vi "TLB Native Dynamic Events ver 0.25.vi"() -> ()   [LabVIEW 2018] (continued)
            n517 = Less?(x=w1477, y=w1481) -> (x < y?=w1480:bool)
            n518 = And(x=w1480, y=w1479) -> (x .and. y?=w1476:bool)
            n519 = case shown="\"Start Task 1\", Default" w1483 {
              tunnel: [w1498 State_Type_Definitions."True Stop" ("Enum")] -> w1488
              tunnel: [w1501 w1518] -> w1487
              tunnel: [State_Type_Definitions."Idle" ("Enum") State_Type_Definitions."Shutdown" ("Enum")] -> w1489
              tunnel: w1491 -> [w1497 _]
              tunnel: w1490 -> [w1493 w1515]
              tunnel: w1476 -> [w1492 _]
              frame "Start Task 1", Default {
                # "Stays in Task 5_B to capture image over 5 seconds"
                # "T: Go back to idle, F: Continue with task\""
                # ">> Manual override >>"
                n520 = case shown="True" w1492 {
                  tunnel: [w1505 w1511] -> w1501
                  tunnel: w1493 -> [w1503 w1509]
                  frame False {
                    n521 = for {
                      tunnel: string[] ["FORWARD", "READ ULTRASONIC", "READ NAVX"] ("element") -> [w1506] mode=indexing
                      shift-right: [w1508] -> w1505
                      shift-left: w1503 -> [w1507]
                      n522 = Enqueue Element(queue=w1507, element=w1506) -> (queue out=w1508:refnum<queue>)  [unwired: 2 in, 2 out]
                    }
                  }
                  frame True {
                    n523 = for {
                      shift-right: [w1513] -> w1511
                      shift-left: w1509 -> [w1514]
                      tunnel: string[] ["STOP", "RESET ENCODERS", "OPEN LOG CAM", "SET TIMER 2", "OPEN IMAQ REF"] -> [w1512] mode=indexing
                      n524 = Enqueue Element(queue=w1514, element=w1512) -> (queue out=w1513:refnum<queue>)  [unwired: 2 in, 2 out]
                    }
                  }
                }
                n525 = Or(x=w1492, y=w1497) -> (x .or. y?=w1499:bool)
                n526 = Select(t=State_Type_Definitions."True Stop" ("Enum"), s=w1497, f=State_Type_Definitions."Task 8C: CAM BURST" ("Enum")) -> (s? t:f=w1494:T16)
                n527 = Select(t=w1494, s=w1499, f=State_Type_Definitions."Task 8B: MOVE TO BOX" ("Enum")) -> (s? t:f=w1498:T16)
              }
              frame "Exit" {
                n528 = for {
                  shift-right: [w1521] -> w1518
                  shift-left: w1515 -> [w1522]
                  tunnel: string[] ["STOP", "RESET ENCODERS", "RESET YAW", "ARDUINO MODE 0"] -> [w1520] mode=indexing
                  n529 = Enqueue Element(queue=w1522, element=w1520) -> (queue out=w1521:refnum<queue>)  [unwired: 2 in, 2 out]
                }
              }
            }
          }
          frame "Task 8C: CAM BURST" {
            # ">>> Motor control cluster >>>"
            # ">>> yStepper command>>>"
            # ">> Manual override >>"
            n530 = Dequeue Element(queue=w1533, timeout in ms (-1)=w1532, error in (no error)=w1531) -> (element=w1530:T8)  [unwired: 3 out]
            n531 = case shown="\"Start Task 1\", Default" w1530 {
              tunnel: [w1542 State_Type_Definitions."True Stop" ("Enum")] -> w1535
              tunnel: [w1545 w1562] -> w1528
              tunnel: [State_Type_Definitions."Idle" ("Enum") State_Type_Definitions."Shutdown" ("Enum")] -> w1527
              tunnel: w1529 -> [w1536 _]
              tunnel: w1534 -> [w1541 w1559]
              tunnel: w1525 -> [w1540 _]
              frame "Start Task 1", Default {
                # ">> Is time up? >>"
                # "Determines if object is in range to pick up"
                # ">> Manual override >>"
                n532 = case shown="True" w1540 {
                  tunnel: [w1549 w1555] -> w1545
                  tunnel: w1541 -> [w1547 w1553]
                  frame False {
                    n533 = for {
                      tunnel: string[] ["CAM ACQ", "START TIMER"] ("element") -> [w1550] mode=indexing
                      shift-right: [w1552] -> w1549
                      shift-left: w1547 -> [w1551]
                      n534 = Enqueue Element(queue=w1551, element=w1550) -> (queue out=w1552:refnum<queue>)  [unwired: 2 in, 2 out]
                    }
                  }
                  frame True {
                    n535 = for {
                      shift-right: [w1557] -> w1555
                      shift-left: w1553 -> [w1558]
                      tunnel: string[] ["CAM CLOSE", "PROCESS IMAGE", "SET TIMER 5"] -> [w1556] mode=indexing
                      n536 = Enqueue Element(queue=w1558, element=w1556) -> (queue out=w1557:refnum<queue>)  [unwired: 2 in, 2 out]
                    }
                  }
                }
                n537 = Or(x=w1540, y=w1536) -> (x .or. y?=w1543:bool)
                n538 = Select(t=State_Type_Definitions."True Stop" ("Enum"), s=w1536, f=State_Type_Definitions."Task 8D: PROCESS IMAGE" ("Enum")) -> (s? t:f=w1538:T16)
                n539 = Select(t=w1538, s=w1543, f=State_Type_Definitions."Task 8C: CAM BURST" ("Enum")) -> (s? t:f=w1542:T16)
              }
              frame "Exit" {
                n540 = for {
                  shift-right: [w1565] -> w1562
                  shift-left: w1559 -> [w1566]
                  tunnel: string[] ["STOP", "RESET ENCODERS", "RESET YAW", "ARDUINO MODE 0"] -> [w1564] mode=indexing
                  n541 = Enqueue Element(queue=w1566, element=w1564) -> (queue out=w1565:refnum<queue>)  [unwired: 2 in, 2 out]
                }
              }
            }
          }
          frame "Task 8D: PROCESS IMAGE" {
            # ">>> yStepper command>>>"
            n542 = Dequeue Element(queue=w1574, timeout in ms (-1)=w1573, error in (no error)=w1572) -> (element=w1571:T8)  [unwired: 3 out]
            n543 = case shown="\"Start Task 1\", Default" w1571 {
              tunnel: [w1586 State_Type_Definitions."True Stop" ("Enum")] -> w1578
              tunnel: [w1589 w1606] -> w1577
              tunnel: [State_Type_Definitions."Idle" ("Enum") State_Type_Definitions."Shutdown" ("Enum")] -> w1579
              tunnel: w1575 -> [w1585 _]
              tunnel: w1576 -> [w1581 w1603]
              tunnel: w1569 -> [w1580 _]
              frame "Start Task 1", Default {
                # ">> T: Breaks out of state loop; F: Stays in loop>>"
                # ">> Manual override >>"
                # ">> Checks if time is up>>"
                # "Stays in Task 5D until the object is detected"
                # "T: Go back to idle, F: Continue with task\""
                # ">> Manual override >>"
                n544 = case shown="True" w1580 {
                  tunnel: [w1593 w1599] -> w1589
                  tunnel: w1581 -> [w1591 w1597]
                  frame False {
                    n545 = for {
                      tunnel: string[] ["START TIMER", "PROCESS IMAGE", ""] ("element") -> [w1594] mode=indexing
                      shift-right: [w1596] -> w1593
                      shift-left: w1591 -> [w1595]
                      n546 = Enqueue Element(queue=w1595, element=w1594) -> (queue out=w1596:refnum<queue>)  [unwired: 2 in, 2 out]
                    }
                  }
                  frame True {
                    n547 = for {
                      shift-right: [w1601] -> w1599
                      shift-left: w1597 -> [w1602]
                      tunnel: string[] ["RESET ENCODERS", "", ""] -> [w1600] mode=indexing
                      n548 = Enqueue Element(queue=w1602, element=w1600) -> (queue out=w1601:refnum<queue>)  [unwired: 2 in, 2 out]
                    }
                  }
                }
                n549 = Or(x=w1580, y=w1585) -> (x .or. y?=w1587:bool)
                n550 = Select(t=State_Type_Definitions."True Stop" ("Enum"), s=w1585, f=State_Type_Definitions."Task 8E: ROBOT ADJUST" ("Enum")) -> (s? t:f=w1582:T16)
                n551 = Select(t=w1582, s=w1587, f=State_Type_Definitions."Task 8D: PROCESS IMAGE" ("Enum")) -> (s? t:f=w1586:T16)
              }
              frame "Exit" {
                n552 = for {
                  shift-right: [w1609] -> w1606
                  shift-left: w1603 -> [w1610]
                  tunnel: string[] ["STOP", "RESET ENCODERS", "RESET YAW", "ARDUINO MODE 0"] -> [w1608] mode=indexing
                  n553 = Enqueue Element(queue=w1610, element=w1608) -> (queue out=w1609:refnum<queue>)  [unwired: 2 in, 2 out]
                }
              }
            }
          }
          frame "Task 8E: ROBOT ADJUST" {
            # ">>> Motor control cluster >>>"
            # ">>> yStepper command>>>"
            n554 = Dequeue Element(queue=w1627, timeout in ms (-1)=w1626, error in (no error)=w1625) -> (element=w1624:T8)  [unwired: 3 out]
            n555 = Subtract(x=w1622, y=300.0) -> (x-y=w1620:dbl)
            n556 = formula code="if (error <= -61&&error > -300){\ndistance = -15;\nxSpeed = -30;\n}\n\nelse if (error <= -51 && error >= -60){\ndistance = -10;\nxSpeed = -30;\n}\n\nelse if (error >= -50 && error <= 50){\ndistance = 0;\nxSpeed = 0;\n}\n\nelse if (error >= 51 && error <= 80){\ndistance = 10;\nxSpeed = 30;\n}\n\nelse if (error >= 81 && error <= 100){\ndistance = 15;\nxSpeed = 30;\n}\n\nelse if (error >= 101 && error <= 120){\ndistance = 20;\nxSpeed = 30;\n}\n\nelse if (error >= 121 && error < 300){\ndistance = 25;\nxSpeed = 30;\n}\n\nelse{\ndistance = 0;\nxSpeed = 0;\n}"("error"=w1620) -> ("distance"=w1615:dbl, "xSpeed"=w1617:dbl)
            n557 = formula code="if (target > 0){\nif (current  >= target)\noutput = 1;\n\nelse if (current != target)\noutput = 0;\n}\n\nelse if (target == 0){\nif (current == target)\noutput = 1;\n\nelse if (current != target)\noutput = 0;\n}\n\nelse if (target < 0){\nif (current <= target)\noutput = 1;\n\nelse if (current != target)\noutput = 0;\n}\n\nelse if (current != target)\noutput = 0;"("target"=w1615, "current"=w1616) -> ("output"=w1614:dbl)
            n558 = Bundle By Name(cluster=w1619, "xSpeed"=w1617) -> (w1618:T17)
            n559 = Equal?(x=w1614, y=1.0) -> (x = y?=w1612:bool)
            n560 = case shown="\"Start Task 1\", Default" w1624 {
              tunnel: [w1639 State_Type_Definitions."True Stop" ("Enum")] -> w1631
              tunnel: [w1642 w1659] -> w1630
              tunnel: [State_Type_Definitions."Idle" ("Enum") State_Type_Definitions."Shutdown" ("Enum")] -> w1632
              tunnel: w1628 -> [w1638 _]
              tunnel: w1629 -> [w1634 w1656]
              tunnel: w1612 -> [w1633 _]
              frame "Start Task 1", Default {
                # ">> T: Breaks out of state loop; F: Stays in loop>>"
                # ">> Manual override >>"
                # ">> Checks if time is up>>"
                # "Stays in Task 5D until the object is detected"
                # "T: Go back to idle, F: Continue with task\""
                # ">> Manual override >>"
                n561 = case shown="True" w1633 {
                  tunnel: [w1646 w1652] -> w1642
                  tunnel: w1634 -> [w1644 w1650]
                  frame False {
                    n562 = for {
                      tunnel: string[] ["X AXIS - SLOW", "READ ENCODERS", "READ NAVX"] ("element") -> [w1647] mode=indexing
                      shift-right: [w1649] -> w1646
                      shift-left: w1644 -> [w1648]
                      n563 = Enqueue Element(queue=w1648, element=w1647) -> (queue out=w1649:refnum<queue>)  [unwired: 2 in, 2 out]
                    }
                  }
                  frame True {
                    n564 = for {
                      shift-right: [w1654] -> w1652
                      shift-left: w1650 -> [w1655]
                      tunnel: string[] ["SET TIMER 2", "STOP", "READ STEPPER VALUES", ""] -> [w1653] mode=indexing
                      n565 = Enqueue Element(queue=w1655, element=w1653) -> (queue out=w1654:refnum<queue>)  [unwired: 2 in, 2 out]
                    }
                  }
                }
                n566 = Or(x=w1633, y=w1638) -> (x .or. y?=w1640:bool)
                n567 = Select(t=State_Type_Definitions."True Stop" ("Enum"), s=w1638, f=State_Type_Definitions."Task 8H: ARM ADJUST" ("Enum")) -> (s? t:f=w1635:T16)
                n568 = Select(t=w1635, s=w1640, f=State_Type_Definitions."Task 8E: ROBOT ADJUST" ("Enum")) -> (s? t:f=w1639:T16)
              }
              frame "Exit" {
                n569 = for {
                  shift-right: [w1662] -> w1659
                  shift-left: w1656 -> [w1663]
                  tunnel: string[] ["STOP", "RESET ENCODERS", "RESET YAW", "ARDUINO MODE 0"] -> [w1661] mode=indexing
                  n570 = Enqueue Element(queue=w1663, element=w1661) -> (queue out=w1662:refnum<queue>)  [unwired: 2 in, 2 out]
                }
              }
            }
          }
          frame "Task 8F: CAM BURST 2" {
            # ">>> Motor control cluster >>>"
            # ">>> yStepper command>>>"
            # ">> Manual override >>"
            n571 = Dequeue Element(queue=w1674, timeout in ms (-1)=w1673, error in (no error)=w1672) -> (element=w1671:T8)  [unwired: 3 out]
            n572 = case shown="\"Start Task 1\", Default" w1671 {
              tunnel: [w1683 State_Type_Definitions."True Stop" ("Enum")] -> w1676
              tunnel: [w1686 w1703] -> w1669
              tunnel: [State_Type_Definitions."Idle" ("Enum") State_Type_Definitions."Shutdown" ("Enum")] -> w1668
              tunnel: w1670 -> [w1677 _]
              tunnel: w1675 -> [w1682 w1700]
              tunnel: w1666 -> [w1681 _]
              frame "Start Task 1", Default {
                # ">> Is time up? >>"
                # "Determines if object is in range to pick up"
                # ">> Manual override >>"
                n573 = case shown="False" w1681 {
                  tunnel: [w1690 w1696] -> w1686
                  tunnel: w1682 -> [w1688 w1694]
                  frame False {
                    n574 = for {
                      tunnel: string[] ["CAM ACQ", "START TIMER"] ("element") -> [w1691] mode=indexing
                      shift-right: [w1693] -> w1690
                      shift-left: w1688 -> [w1692]
                      n575 = Enqueue Element(queue=w1692, element=w1691) -> (queue out=w1693:refnum<queue>)  [unwired: 2 in, 2 out]
                    }
                  }
                  frame True {
                    n576 = for {
                      shift-right: [w1698] -> w1696
                      shift-left: w1694 -> [w1699]
                      tunnel: string[] ["CAM CLOSE", "PROCESS IMAGE", "SET TIMER 3"] -> [w1697] mode=indexing
                      n577 = Enqueue Element(queue=w1699, element=w1697) -> (queue out=w1698:refnum<queue>)  [unwired: 2 in, 2 out]
                    }
                  }
                }
                n578 = Or(x=w1681, y=w1677) -> (x .or. y?=w1684:bool)
                n579 = Select(t=State_Type_Definitions."True Stop" ("Enum"), s=w1677, f=State_Type_Definitions."Task 8G: PROCESS IMAGE 2" ("Enum")) -> (s? t:f=w1679:T16)
                n580 = Select(t=w1679, s=w1684, f=State_Type_Definitions."Task 8F: CAM BURST 2" ("Enum")) -> (s? t:f=w1683:T16)
              }
              frame "Exit" {
                n581 = for {
                  shift-right: [w1706] -> w1703
                  shift-left: w1700 -> [w1707]
                  tunnel: string[] ["STOP", "RESET ENCODERS", "RESET YAW", "ARDUINO MODE 0"] -> [w1705] mode=indexing
                  n582 = Enqueue Element(queue=w1707, element=w1705) -> (queue out=w1706:refnum<queue>)  [unwired: 2 in, 2 out]
                }
              }
            }
          }
          frame "Task 8G: PROCESS IMAGE 2" {
            # ">>> yStepper command>>>"
            n583 = Dequeue Element(queue=w1715, timeout in ms (-1)=w1714, error in (no error)=w1713) -> (element=w1712:T8)  [unwired: 3 out]
            n584 = case shown="\"Start Task 1\", Default" w1712 {
              tunnel: [w1727 State_Type_Definitions."True Stop" ("Enum")] -> w1719
              tunnel: [w1730 w1747] -> w1718
              tunnel: [State_Type_Definitions."Idle" ("Enum") State_Type_Definitions."Shutdown" ("Enum")] -> w1720
              tunnel: w1716 -> [w1726 _]
              tunnel: w1717 -> [w1722 w1744]
              tunnel: w1710 -> [w1721 _]
              frame "Start Task 1", Default {
                # ">> T: Breaks out of state loop; F: Stays in loop>>"
                # ">> Manual override >>"
                # ">> Checks if time is up>>"
                # "Stays in Task 5D until the object is detected"
                # "T: Go back to idle, F: Continue with task\""
                # ">> Manual override >>"
                n585 = case shown="False" w1721 {
                  tunnel: [w1734 w1740] -> w1730
                  tunnel: w1722 -> [w1732 w1738]
                  frame False {
                    n586 = for {
                      tunnel: string[] ["START TIMER", "PROCESS IMAGE", ""] ("element") -> [w1735] mode=indexing
                      shift-right: [w1737] -> w1734
                      shift-left: w1732 -> [w1736]
                      n587 = Enqueue Element(queue=w1736, element=w1735) -> (queue out=w1737:refnum<queue>)  [unwired: 2 in, 2 out]
                    }
                  }
                  frame True {
                    n588 = for {
                      shift-right: [w1742] -> w1740
                      shift-left: w1738 -> [w1743]
                      tunnel: string[] ["READ STEPPER VALUES", "Y STEPPER CONTROL", ""] -> [w1741] mode=indexing
                      n589 = Enqueue Element(queue=w1743, element=w1741) -> (queue out=w1742:refnum<queue>)  [unwired: 2 in, 2 out]
                    }
                  }
                }
                n590 = Or(x=w1721, y=w1726) -> (x .or. y?=w1728:bool)
                n591 = Select(t=State_Type_Definitions."True Stop" ("Enum"), s=w1726, f=State_Type_Definitions."Task 8H: ARM ADJUST" ("Enum")) -> (s? t:f=w1723:T16)
                n592 = Select(t=w1723, s=w1728, f=State_Type_Definitions."Task 8G: PROCESS IMAGE 2" ("Enum")) -> (s? t:f=w1727:T16)
              }
              frame "Exit" {
                n593 = for {
                  shift-right: [w1750] -> w1747
                  shift-left: w1744 -> [w1751]
                  tunnel: string[] ["STOP", "RESET ENCODERS", "RESET YAW", "ARDUINO MODE 0"] -> [w1749] mode=indexing
                  n594 = Enqueue Element(queue=w1751, element=w1749) -> (queue out=w1750:refnum<queue>)  [unwired: 2 in, 2 out]
                }
              }
            }
          }
          frame "Task 8H: ARM ADJUST" {
            # ">>> yStepper command>>>"
            n595 = Dequeue Element(queue=w1765, timeout in ms (-1)=w1766, error in (no error)=w1767) -> (element=w1769:T8)  [unwired: 3 out]
            n596 = formula code="if (pos < 70)\ny = 43;\n\nelse if (pos >= 71 &&pos <= 80)\ny = 40;\n\nelse if (pos >= 81 && pos <= 90)\ny = 38;\n\nelse if (pos >= 91 &&pos <= 120)\ny = 35;\n\nelse if (pos >= 121 && pos <= 140)\ny = 30;\n\nelse if (pos >= 141 && pos <= 170)\ny = 26;\n\nelse if (pos >= 171 &&pos <= 220) \ny = 20;\n\nelse if (pos >= 221&& pos <= 240)\ny = 15;\n\nelse if (pos >= 241 && pos <= 250)\ny = 10;\n\nelse if (pos >= 251)\ny = 0;"("pos"=w1757) -> ("y"=w1760:dbl)
            n597 = To Unsigned Byte Integer(number=w1760) -> (unsigned 8bit integer=w1755:u8)
            n598 = Equal?(x=w1756, y=w1755) -> (x = y?=w1754:bool)
            n599 = case shown="\"Start Task 1\", Default" w1769 {
              tunnel: [w1776 State_Type_Definitions."True Stop" ("Enum")] -> w1763
              tunnel: [w1779 w1796] -> w1761
              tunnel: [State_Type_Definitions."Idle" ("Enum") State_Type_Definitions."Shutdown" ("Enum")] -> w1762
              tunnel: w1768 -> [w1775 _]
              tunnel: w1764 -> [w1771 w1793]
              tunnel: w1754 -> [w1770 _]
              frame "Start Task 1", Default {
                # ">> T: Breaks out of state loop; F: Stays in loop>>"
                # ">> Manual override >>"
                # ">> Checks if time is up>>"
                # "Stays in Task 5D until the object is detected"
                # "T: Go back to idle, F: Continue with task\""
                # ">> Manual override >>"
                n600 = case shown="False" w1770 {
                  tunnel: [w1783 w1789] -> w1779
                  tunnel: w1771 -> [w1781 w1787]
                  frame False {
                    n601 = for {
                      tunnel: string[] ["READ STEPPER VALUES", "Y STEPPER CONTROL", ""] ("element") -> [w1784] mode=indexing
                      shift-right: [w1786] -> w1783
                      shift-left: w1781 -> [w1785]
                      n602 = Enqueue Element(queue=w1785, element=w1784) -> (queue out=w1786:refnum<queue>)  [unwired: 2 in, 2 out]
                    }
                  }
                  frame True {
                    n603 = for {
                      shift-right: [w1791] -> w1789
                      shift-left: w1787 -> [w1792]
                      tunnel: string[] ["DISPOSE BUFFERS", "READ STEPPER VALUES", ""] -> [w1790] mode=indexing
                      n604 = Enqueue Element(queue=w1792, element=w1790) -> (queue out=w1791:refnum<queue>)  [unwired: 2 in, 2 out]
                    }
                  }
                }
                n605 = Or(x=w1770, y=w1775) -> (x .or. y?=w1777:bool)
                n606 = Select(t=State_Type_Definitions."True Stop" ("Enum"), s=w1775, f=State_Type_Definitions."Task 8I: ARM GRAB HEIGHT" ("Enum")) -> (s? t:f=w1772:T16)
                n607 = Select(t=w1772, s=w1777, f=State_Type_Definitions."Task 8H: ARM ADJUST" ("Enum")) -> (s? t:f=w1776:T16)
              }
              frame "Exit" {
                n608 = for {
                  shift-right: [w1799] -> w1796
                  shift-left: w1793 -> [w1800]
                  tunnel: string[] ["STOP", "RESET ENCODERS", "RESET YAW", "ARDUINO MODE 0"] -> [w1798] mode=indexing
                  n609 = Enqueue Element(queue=w1800, element=w1798) -> (queue out=w1799:refnum<queue>)  [unwired: 2 in, 2 out]
                }
              }
            }
            n610 = Bundle By Name(cluster=w1759, "yStepper desired"=w1755) -> (w1758:T18)
          }
          frame "Task 8I: ARM GRAB HEIGHT" {
            # ">>> Motor control cluster >>>"
            # ">>> yStepper command>>>"
            # ">> Manual override >>"
            n611 = Dequeue Element(queue=w1811, timeout in ms (-1)=w1810, error in (no error)=w1812) -> (element=w1809:T8)  [unwired: 3 out]
            n612 = Equal?(x=w1808, y=u8 1) -> (x = y?=w1806:bool)
            n613 = case shown="\"Start Task 1\", Default" w1809 {
              tunnel: [w1822 State_Type_Definitions."True Stop" ("Enum")] -> w1813
              tunnel: [w1825 w1842] -> w1814
              tunnel: [State_Type_Definitions."Idle" ("Enum") State_Type_Definitions."Shutdown" ("Enum")] -> w1815
              tunnel: w1806 -> [w1821 _]
              tunnel: w1805 -> [w1820 _]
              tunnel: w1804 -> [w1816 w1839]
              frame "Start Task 1", Default {
                # "Stays in Task 5F until stepper reaches desired \nheight"
                # "T: Go back to idle, F: Continue with task\""
                # ">> Manual override >>"
                n614 = case shown="True" w1821 {
                  tunnel: [w1829 w1835] -> w1825
                  tunnel: w1816 -> [w1827 w1833]
                  frame False {
                    n615 = for {
                      tunnel: string[] ["Z STEPPER GRAB HEIGHT", "READ STEPPER VALUES"] ("element") -> [w1830] mode=indexing
                      shift-right: [w1832] -> w1829
                      shift-left: w1827 -> [w1831]
                      n616 = Enqueue Element(queue=w1831, element=w1830) -> (queue out=w1832:refnum<queue>)  [unwired: 2 in, 2 out]
                    }
                  }
                  frame True {
                    n617 = for {
                      shift-right: [w1837] -> w1835
                      shift-left: w1833 -> [w1838]
                      tunnel: string[] ["SET TIMER 2", "CLOSE CLAW", ""] -> [w1836] mode=indexing
                      n618 = Enqueue Element(queue=w1838, element=w1836) -> (queue out=w1837:refnum<queue>)  [unwired: 2 in, 2 out]
                    }
                  }
                }
                n619 = Or(x=w1821, y=w1820) -> (x .or. y?=w1823:bool)
                n620 = Select(t=State_Type_Definitions."True Stop" ("Enum"), s=w1820, f=State_Type_Definitions."Task 8J: CLOSE CLAW" ("Enum")) -> (s? t:f=w1817:T16)
                n621 = Select(t=w1817, s=w1823, f=State_Type_Definitions."Task 8I: ARM GRAB HEIGHT" ("Enum")) -> (s? t:f=w1822:T16)
              }
              frame "Exit" {
                n622 = for {
                  shift-right: [w1845] -> w1842
                  shift-left: w1839 -> [w1846]
                  tunnel: string[] ["STOP", "RESET ENCODERS", "RESET YAW", "ARDUINO MODE 0"] -> [w1844] mode=indexing
                  n623 = Enqueue Element(queue=w1846, element=w1844) -> (queue out=w1845:refnum<queue>)  [unwired: 2 in, 2 out]
                }
              }
            }
          }
          frame "Task 8J: CLOSE CLAW" {
            # ">>> yStepper command>>>"
            # ">> Manual override >>"
            n624 = Dequeue Element(queue=w1857, timeout in ms (-1)=w1856, error in (no error)=w1855) -> (element=w1854:T8)  [unwired: 3 out]
            n625 = case shown="\"Start Task 1\", Default" w1854 {
              tunnel: [w1866 State_Type_Definitions."True Stop" ("Enum")] -> w1859
              tunnel: [w1869 w1886] -> w1852
              tunnel: [State_Type_Definitions."Idle" ("Enum") State_Type_Definitions."Shutdown" ("Enum")] -> w1851
              tunnel: w1853 -> [w1860 _]
              tunnel: w1858 -> [w1865 w1883]
              tunnel: w1849 -> [w1864 _]
              frame "Start Task 1", Default {
                # ">> Is time up? >>"
                # "Determines if object is in range to pick up"
                # ">> Manual override >>"
                n626 = case shown="True" w1864 {
                  tunnel: [w1873 w1879] -> w1869
                  tunnel: w1865 -> [w1871 w1877]
                  frame False {
                    n627 = for {
                      tunnel: string[] ["CLOSE CLAW", "START TIMER"] ("element") -> [w1874] mode=indexing
                      shift-right: [w1876] -> w1873
                      shift-left: w1871 -> [w1875]
                      n628 = Enqueue Element(queue=w1875, element=w1874) -> (queue out=w1876:refnum<queue>)  [unwired: 2 in, 2 out]
                    }
                  }
                  frame True {
                    n629 = for {
                      shift-right: [w1881] -> w1879
                      shift-left: w1877 -> [w1882]
                      tunnel: string[] ["READ STEPPER VALUES", "", ""] -> [w1880] mode=indexing
                      n630 = Enqueue Element(queue=w1882, element=w1880) -> (queue out=w1881:refnum<queue>)  [unwired: 2 in, 2 out]
                    }
                  }
                }
                n631 = Or(x=w1864, y=w1860) -> (x .or. y?=w1867:bool)
                n632 = Select(t=State_Type_Definitions."True Stop" ("Enum"), s=w1860, f=State_Type_Definitions."Task 8K: RAISE MY SWORD" ("Enum")) -> (s? t:f=w1862:T16)
                n633 = Select(t=w1862, s=w1867, f=State_Type_Definitions."Task 8J: CLOSE CLAW" ("Enum")) -> (s? t:f=w1866:T16)
              }
              frame "Exit" {
                n634 = for {
                  shift-right: [w1889] -> w1886
                  shift-left: w1883 -> [w1890]
                  tunnel: string[] ["STOP", "RESET ENCODERS", "RESET YAW", "ARDUINO MODE 0"] -> [w1888] mode=indexing
                  n635 = Enqueue Element(queue=w1890, element=w1888) -> (queue out=w1889:refnum<queue>)  [unwired: 2 in, 2 out]
                }
              }
            }
          }
          frame "Task 8K: RAISE MY SWORD" {
            # ">>> yStepper command>>>"
            # ">> Manual override >>"
            n636 = Dequeue Element(queue=w1901, timeout in ms (-1)=w1900, error in (no error)=w1902) -> (element=w1899:T8)  [unwired: 3 out]
            n637 = Equal?(x=w1898, y=u8 60) -> (x = y?=w1896:bool)
            n638 = case shown="\"Start Task 1\", Default" w1899 {
              tunnel: [w1912 State_Type_Definitions."True Stop" ("Enum")] -> w1903
              tunnel: [w1915 w1932] -> w1904
              tunnel: [State_Type_Definitions."Idle" ("Enum") State_Type_Definitions."Shutdown" ("Enum")] -> w1905
              tunnel: w1896 -> [w1911 _]
              tunnel: w1895 -> [w1910 _]
              tunnel: w1894 -> [w1906 w1929]
              frame "Start Task 1", Default {
                # "Stays in Task 5_A until stepper reaches desired \nheight"
                # "T: Go back to idle, F: Continue with task\""
                # ">> Manual override >>"
                n639 = case shown="True" w1911 {
                  tunnel: [w1919 w1925] -> w1915
                  tunnel: w1906 -> [w1917 w1923]
                  frame False {
                    n640 = for {
                      tunnel: string[] ["Z STEPPER CAM HEIGHT", "READ STEPPER VALUES"] ("element") -> [w1920] mode=indexing
                      shift-right: [w1922] -> w1919
                      shift-left: w1917 -> [w1921]
                      n641 = Enqueue Element(queue=w1921, element=w1920) -> (queue out=w1922:refnum<queue>)  [unwired: 2 in, 2 out]
                    }
                  }
                  frame True {
                    n642 = for {
                      shift-right: [w1927] -> w1925
                      shift-left: w1923 -> [w1928]
                      tunnel: string[] ["CAM CLOSE", "DISPOSE CAM BUFFERS", "DISPOSE PROC BUFFERS", "RESET ENCODERS"] -> [w1926] mode=indexing
                      n643 = Enqueue Element(queue=w1928, element=w1926) -> (queue out=w1927:refnum<queue>)  [unwired: 2 in, 2 out]
                    }
                  }
                }
                n644 = Or(x=w1911, y=w1910) -> (x .or. y?=w1913:bool)
                n645 = Select(t=State_Type_Definitions."True Stop" ("Enum"), s=w1910, f=State_Type_Definitions."True Stop" ("Enum")) -> (s? t:f=w1907:T16)
                n646 = Select(t=w1907, s=w1913, f=State_Type_Definitions."Task 8K: RAISE MY SWORD" ("Enum")) -> (s? t:f=w1912:T16)
              }
              frame "Exit" {
                n647 = for {
                  shift-right: [w1935] -> w1932
                  shift-left: w1929 -> [w1936]
                  tunnel: string[] ["STOP", "RESET ENCODERS", "RESET YAW", "ARDUINO MODE 0"] -> [w1934] mode=indexing
                  n648 = Enqueue Element(queue=w1936, element=w1934) -> (queue out=w1935:refnum<queue>)  [unwired: 2 in, 2 out]
                }
              }
            }
          }
          frame "Task 9A: Raise Arm" {
            # ">>> Motor control cluster >>>"
            # ">> Stepper height reeached >>"
            # ">>> yStepper command>>>"
            # ">> Manual override >>"
            n649 = Dequeue Element(queue=w1948, timeout in ms (-1)=w1943, error in (no error)=w1947) -> (element=w1951:T8)  [unwired: 3 out]
            n650 = Equal?(x=w1945, y=u8 40) -> (x = y?=w1949:bool)
            n651 = case shown="\"Start Task 1\", Default" w1951 {
              tunnel: [w1962 State_Type_Definitions."True Stop" ("Enum")] -> w1941
              tunnel: [w1960 w1977] -> w1940
              tunnel: w1944 -> [w1959 _]
              tunnel: w1946 -> [w1953 _]
              tunnel: [State_Type_Definitions."Idle" ("Enum") State_Type_Definitions."Shutdown" ("Enum")] -> w1942
              tunnel: w1949 -> [w1952 _]
              frame "Start Task 1", Default {
                # ">> WIill proceed to part ii if not manual override >>"
                # ">>If ENABLE or Trigger is set to true>>"
                n652 = Or(x=w1952, y=w1953) -> (x .or. y?=w1954:bool)
                n653 = case shown="True" w1952 {
                  tunnel: [w1965 w1971] -> w1960
                  tunnel: w1959 -> [w1964 w1970]
                  frame False {
                    n654 = for {
                      shift-right: [w1967] -> w1965
                      shift-left: w1964 -> [w1968]
                      tunnel: string[] ["Z STEPPER BOX HEIGHT", "READ STEPPER VALUES"] ("element") -> [w1966] mode=indexing
                      n655 = Enqueue Element(queue=w1968, element=w1966) -> (queue out=w1967:refnum<queue>)  [unwired: 2 in, 2 out]
                    }
                  }
                  frame True {
                    n656 = for {
                      shift-right: [w1973] -> w1971
                      shift-left: w1970 -> [w1974]
                      tunnel: string[] ["ARDUINO - ULTRASONIC", "READ NAVX", "RESET FLAGS", "", "", ""] -> [w1972] mode=indexing
                      n657 = Enqueue Element(queue=w1974, element=w1972) -> (queue out=w1973:refnum<queue>)  [unwired: 2 in, 2 out]
                    }
                  }
                }
                n658 = Select(t=State_Type_Definitions."True Stop" ("Enum"), s=w1953, f=State_Type_Definitions."Task 9B: Rotate to Angle" ("Enum")) -> (s? t:f=w1956:T16)
                n659 = Select(t=w1956, s=w1954, f=State_Type_Definitions."Task 9A: Raise Arm" ("Enum")) -> (s? t:f=w1962:T16)
              }
              frame "Exit" {
                n660 = for {
                  shift-right: [w1980] -> w1977
                  shift-left: _ -> [w1981]
                  tunnel: string[] ["STOP", "RESET ENCODERS", "RESET YAW", ""] -> [w1979] mode=indexing
                  n661 = Enqueue Element(queue=w1981, element=w1979) -> (queue out=w1980:refnum<queue>)  [unwired: 2 in, 2 out]
                }
              }
            }
          }
          frame "Task 9B: Rotate to Angle" {
            # ">>> Motor control cluster >>>"
            # ">>> yStepper command>>>"
            n662 = Dequeue Element(queue=w1995, timeout in ms (-1)=w1994, error in (no error)=w1993) -> (element=w1997:T8)  [unwired: 3 out]
            n663 = In Range and Coerce(upper limit=65.0, x=w1987, lower limit=55.0) -> (In Range?=w1984:bool)  [unwired: 1 out]
            n664 = case shown="\"Start Task 1\", Default" w1997 {
              tunnel: w1988 -> [w2000 _]
              tunnel: [w2008 State_Type_Definitions."True Stop" ("Enum")] -> w1990
              tunnel: w1996 -> [w2006 w2024]
              tunnel: [w2005 w2023] -> w1989
              tunnel: [State_Type_Definitions."Idle" ("Enum") State_Type_Definitions."Shutdown" ("Enum")] -> w1991
              tunnel: w1984 -> [w1998 _]
              frame "Start Task 1", Default {
                n665 = Or(x=w1998, y=w2000) -> (x .or. y?=w1999:bool)
                n666 = case shown="True" w1998 {
                  tunnel: w2006 -> [w2011 w2017]
                  tunnel: [w2010 w2015] -> w2005
                  frame False {
                    n667 = for {
                      shift-right: [w2013] -> w2010
                      shift-left: w2011 -> [w2014]
                      tunnel: string[] ["READ NAVX", "R-CW", "READ ULTRASONIC"] ("element") -> [w2012] mode=indexing
                      n668 = Enqueue Element(queue=w2014, element=w2012) -> (queue out=w2013:refnum<queue>)  [unwired: 2 in, 2 out]
                    }
                  }
                  frame True {
                    n669 = for {
                      shift-right: [w2019] -> w2015
                      shift-left: w2017 -> [w2020]
                      tunnel: string[] ["STOP", "RESET ENCODERS", "RESET YAW", "ARDUINO - ULTRASONIC", ""] -> [w2018] mode=indexing
                      n670 = Enqueue Element(queue=w2020, element=w2018) -> (queue out=w2019:refnum<queue>)  [unwired: 2 in, 2 out]
                    }
                  }
                }
                n671 = Select(t=State_Type_Definitions."True Stop" ("Enum"), s=w2000, f=State_Type_Definitions."Task 9C: Detect Box") -> (s? t:f=w2002:T16)
                n672 = Select(t=w2002, s=w1999, f=State_Type_Definitions."Task 9B: Rotate to Angle" ("Enum")) -> (s? t:f=w2008:T16)
              }
              frame "Exit" {
                n673 = for {
                  shift-right: [w2027] -> w2023
                  shift-left: w2024 -> [w2028]
                  tunnel: string[] ["STOP", "RESET ENCODERS", "RESET YAW", ""] -> [w2026] mode=indexing
                  n674 = Enqueue Element(queue=w2028, element=w2026) -> (queue out=w2027:refnum<queue>)  [unwired: 2 in, 2 out]
                }
              }
            }
          }
          frame "Task 9C: Detect Box" {
            # ">>> Motor control cluster >>>"
            # ">>Line Detected>>"
            # ">>Action Queue>>"
            # ">>> yStepper command>>>"
            n675 = Dequeue Element(queue=w2040, timeout in ms (-1)=w2039, error in (no error)=w2038) -> (element=w2041:T8)  [unwired: 3 out]
            n676 = case shown="\"Start Task 1\", Default" w2041 {
              tunnel: w2036 -> [w2042 _]
              tunnel: [w2052 State_Type_Definitions."True Stop" ("Enum")] -> w2033
              tunnel: w2037 -> [w2050 w2068]
              tunnel: [w2049 w2067] -> w2032
              tunnel: [State_Type_Definitions."Idle" ("Enum") State_Type_Definitions."Shutdown" ("Enum")] -> w2035
              tunnel: w2030 -> [w2043 _]
              frame "Start Task 1", Default {
                n677 = Or(x=w2042, y=w2043) -> (x .or. y?=w2044:bool)
                n678 = case shown="True" w2043 {
                  tunnel: w2050 -> [w2055 w2061]
                  tunnel: [w2054 w2059] -> w2049
                  frame False {
                    n679 = for {
                      shift-right: [w2057] -> w2054
                      shift-left: w2055 -> [w2058]
                      tunnel: string[] ["READ IR", "READ LINE SENSOR", "FORWARD - IR ASSIST"] ("element") -> [w2056] mode=indexing
                      n680 = Enqueue Element(queue=w2058, element=w2056) -> (queue out=w2057:refnum<queue>)  [unwired: 2 in, 2 out]
                    }
                  }
                  frame True {
                    n681 = for {
                      shift-right: [w2063] -> w2059
                      shift-left: w2061 -> [w2064]
                      tunnel: string[] ["STOP", "RESET ENCODERS", "RESET YAW", ""] -> [w2062] mode=indexing
                      n682 = Enqueue Element(queue=w2064, element=w2062) -> (queue out=w2063:refnum<queue>)  [unwired: 2 in, 2 out]
                    }
                  }
                }
                n683 = Select(t=State_Type_Definitions."True Stop" ("Enum"), s=w2042, f=State_Type_Definitions."Task 9D: MOVE FORWARD") -> (s? t:f=w2046:T16)
                n684 = Select(t=w2046, s=w2044, f=State_Type_Definitions."Task 9C: Detect Box" ("Enum")) -> (s? t:f=w2052:T16)
              }
              frame "Exit" {
                n685 = for {
                  shift-right: [w2071] -> w2067
                  shift-left: w2068 -> [w2072]
                  tunnel: string[] ["STOP", "RESET ENCODERS", "RESET YAW", ""] -> [w2070] mode=indexing
                  n686 = Enqueue Element(queue=w2072, element=w2070) -> (queue out=w2071:refnum<queue>)  [unwired: 2 in, 2 out]
                }
              }
            }
          }
          frame "Task 9D: MOVE FORWARD" {
            # ">> Item Selection Bias >>"
            # ">> Wall detected >>"
            # ">> Manual override >>"
            # ">>Table Detected>>"
            # ">>> Motor control cluster >>>"
            # ">>Table or wall detectected>>"
            # ">>Action Queue>>"
            # ">>> yStepper command>>>"
            n687 = Less Or Equal?(x=w2079, y=15.0) -> (x <= y?=w2073:bool)
            n688 = Less?(x=w2076, y=100.0) -> (x < y?=w2074:bool)
            n689 = Dequeue Element(queue=w2090, timeout in ms (-1)=w2089, error in (no error)=w2088) -> (element=w2091:T8)  [unwired: 3 out]
            n690 = Or(x=w2073, y=w2074) -> (x .or. y?=w2077:bool)
            n691 = case shown="\"Start Task 1\", Default" w2091 {
              tunnel: w2086 -> [w2092 _]
              tunnel: [w2102 State_Type_Definitions."True Stop" ("Enum")] -> w2083
              tunnel: w2087 -> [w2100 w2118]
              tunnel: [w2099 w2117] -> w2082
              tunnel: [State_Type_Definitions."Idle" ("Enum") State_Type_Definitions."Shutdown" ("Enum")] -> w2085
              tunnel: w2077 -> [w2093 _]
              frame "Start Task 1", Default {
                n692 = Or(x=w2092, y=w2093) -> (x .or. y?=w2094:bool)
                n693 = case shown="False" w2093 {
                  tunnel: w2100 -> [w2105 w2111]
                  tunnel: [w2104 w2109] -> w2099
                  frame False {
                    n694 = for {
                      shift-right: [w2107] -> w2104
                      shift-left: w2105 -> [w2108]
                      tunnel: string[] ["READ IR", "FORWARD - IR ASSIST", "READ ULTRASONIC"] ("element") -> [w2106] mode=indexing
                      n695 = Enqueue Element(queue=w2108, element=w2106) -> (queue out=w2107:refnum<queue>)  [unwired: 2 in, 2 out]
                    }
                  }
                  frame True {
                    n696 = for {
                      shift-right: [w2113] -> w2109
                      shift-left: w2111 -> [w2114]
                      tunnel: string[] ["STOP", "RESET ENCODERS", "RESET YAW", ""] -> [w2112] mode=indexing
                      n697 = Enqueue Element(queue=w2114, element=w2112) -> (queue out=w2113:refnum<queue>)  [unwired: 2 in, 2 out]
                    }
                  }
                }
                n698 = Select(t=State_Type_Definitions."True Stop" ("Enum"), s=w2092, f=State_Type_Definitions."True Stop") -> (s? t:f=w2096:T16)
                n699 = Select(t=w2096, s=w2094, f=State_Type_Definitions."Task 9D: MOVE FORWARD" ("Enum")) -> (s? t:f=w2102:T16)
              }
              frame "Exit" {
                n700 = for {
                  shift-right: [w2121] -> w2117
                  shift-left: w2118 -> [w2122]
                  tunnel: string[] ["STOP", "RESET ENCODERS", "RESET YAW", ""] -> [w2120] mode=indexing
                  n701 = Enqueue Element(queue=w2122, element=w2120) -> (queue out=w2121:refnum<queue>)  [unwired: 2 in, 2 out]
                }
              }
            }
          }
          frame "Task 9E: MOVE LEFT" {
            # ">> Item Selection Bias >>"
            # ">> Line detected? >>"
            # ">> Manual override >>"
            # ">>> Motor control cluster >>>"
            # ">>Action Queue>>"
            # ">>> yStepper command>>>"
            n702 = Dequeue Element(queue=w2134, timeout in ms (-1)=w2133, error in (no error)=w2132) -> (element=w2135:T8)  [unwired: 3 out]
            n703 = case shown="\"Start Task 1\", Default" w2135 {
              tunnel: w2130 -> [w2136 _]
              tunnel: [w2146 State_Type_Definitions."True Stop" ("Enum")] -> w2127
              tunnel: w2131 -> [w2144 w2162]
              tunnel: [w2143 w2161] -> w2126
              tunnel: [State_Type_Definitions."Idle" ("Enum") State_Type_Definitions."Shutdown" ("Enum")] -> w2129
              tunnel: w2123 -> [w2137 _]
              frame "Start Task 1", Default {
                n704 = Or(x=w2136, y=w2137) -> (x .or. y?=w2138:bool)
                n705 = case shown="False" w2137 {
                  tunnel: w2144 -> [w2149 w2155]
                  tunnel: [w2148 w2153] -> w2143
                  frame False {
                    n706 = for {
                      shift-right: [w2151] -> w2148
                      shift-left: w2149 -> [w2152]
                      tunnel: string[] ["LEFT", "READ NAVX", "READ LINE SENSOR", ""] ("element") -> [w2150] mode=indexing
                      n707 = Enqueue Element(queue=w2152, element=w2150) -> (queue out=w2151:refnum<queue>)  [unwired: 2 in, 2 out]
                    }
                  }
                  frame True {
                    n708 = for {
                      shift-right: [w2157] -> w2153
                      shift-left: w2155 -> [w2158]
                      tunnel: string[] ["STOP", "RESET ENCODERS", "RESET YAW", "RESET FLAGS", "OPEN LIFE CAM", "SET TIMER 2"] -> [w2156] mode=indexing
                      n709 = Enqueue Element(queue=w2158, element=w2156) -> (queue out=w2157:refnum<queue>)  [unwired: 2 in, 2 out]
                    }
                  }
                }
                n710 = Select(t=State_Type_Definitions."True Stop" ("Enum"), s=w2136, f=State_Type_Definitions."Task 9F: SCAN IMAGE") -> (s? t:f=w2140:T16)
                n711 = Select(t=w2140, s=w2138, f=State_Type_Definitions."Task 9E: MOVE LEFT" ("Enum")) -> (s? t:f=w2146:T16)
              }
              frame "Exit" {
                n712 = for {
                  shift-right: [w2165] -> w2161
                  shift-left: w2162 -> [w2166]
                  tunnel: string[] ["STOP", "RESET ENCODERS", "RESET YAW", ""] -> [w2164] mode=indexing
                  n713 = Enqueue Element(queue=w2166, element=w2164) -> (queue out=w2165:refnum<queue>)  [unwired: 2 in, 2 out]
                }
              }
            }
          }
          frame "Task 9F: SCAN IMAGE" {
            # ">>> Motor control cluster >>>"
            # ">>Time up? >>"
            # ">>> yStepper command>>>"
            # ">> Manual override >>"
            n714 = Dequeue Element(queue=w2178, timeout in ms (-1)=w2174, error in (no error)=w2177) -> (element=w2179:T8)  [unwired: 3 out]
            n715 = case shown="\"Start Task 1\", Default" w2179 {
              tunnel: [w2190 State_Type_Definitions."True Stop" ("Enum")] -> w2172
              tunnel: [w2188 w2206] -> w2171
              tunnel: w2175 -> [w2187 w2203]
              tunnel: w2176 -> [w2181 _]
              tunnel: [State_Type_Definitions."Idle" ("Enum") State_Type_Definitions."Shutdown" ("Enum")] -> w2173
              tunnel: w2167 -> [w2180 _]
              frame "Start Task 1", Default {
                # ">> WIill proceed to part ii if not manual override >>"
                # ">>If ENABLE or Trigger is set to true>>"
                n716 = Or(x=w2180, y=w2181) -> (x .or. y?=w2182:bool)
                n717 = case shown="True" w2180 {
                  tunnel: [w2193 w2199] -> w2188
                  tunnel: w2187 -> [w2192 w2198]
                  frame False {
                    n718 = for {
                      shift-right: [w2195] -> w2193
                      shift-left: w2192 -> [w2196]
                      tunnel: string[] ["CAM ACQ", "START TIMER"] ("element") -> [w2194] mode=indexing
                      n719 = Enqueue Element(queue=w2196, element=w2194) -> (queue out=w2195:refnum<queue>)  [unwired: 2 in, 2 out]
                    }
                  }
                  frame True {
                    n720 = for {
                      shift-right: [w2201] -> w2199
                      shift-left: w2198 -> [w2202]
                      tunnel: string[] ["CLOSE CAM", "SET TIMER 5", "", "", "", ""] -> [w2200] mode=indexing
                      n721 = Enqueue Element(queue=w2202, element=w2200) -> (queue out=w2201:refnum<queue>)  [unwired: 2 in, 2 out]
                    }
                  }
                }
                n722 = Select(t=State_Type_Definitions."True Stop" ("Enum"), s=w2181, f=State_Type_Definitions."Task 9G: PROCESS COLOUR" ("Enum")) -> (s? t:f=w2184:T16)
                n723 = Select(t=w2184, s=w2182, f=State_Type_Definitions."Task 9F: SCAN IMAGE" ("Enum")) -> (s? t:f=w2190:T16)
              }
              frame "Exit" {
                n724 = for {
                  shift-right: [w2209] -> w2206
                  shift-left: w2203 -> [w2210]
                  tunnel: string[] ["STOP", "RESET ENCODERS", "RESET YAW", ""] -> [w2208] mode=indexing
                  n725 = Enqueue Element(queue=w2210, element=w2208) -> (queue out=w2209:refnum<queue>)  [unwired: 2 in, 2 out]
                }
              }
            }
          }
          frame "Task 9G: PROCESS COLOUR" {
            # ">>> Motor control cluster >>>"
            # ">>> yStepper command>>>"
            # ">>Object detected>>"
            n726 = Less Or Equal?(x=w2214, y=30.0) -> (x <= y?=w2212:bool)
            "Table obstruct" <- w2212
            n727 = Dequeue Element(queue=w2220, timeout in ms (-1)=w2219, error in (no error)=w2218) -> (element=w2225:T8)  [unwired: 3 out]
            n728 = case shown="\"Start Task 1\", Default" w2225 {
              tunnel: w2212 -> [w2228 _]
              tunnel: [w2235 State_Type_Definitions."True Stop" ("Enum")] -> w2224
              tunnel: w2217 -> [w2227 _]
              tunnel: w2221 -> [w2234 w2251]
              tunnel: [w2233 w2252] -> w2223
              tunnel: [State_Type_Definitions."Idle" ("Enum") State_Type_Definitions."Shutdown" ("Enum")] -> w2222
              frame "Start Task 1", Default {
                n729 = case shown="True" w2228 {
                  tunnel: w2234 -> [w2238 w2245]
                  tunnel: [w2239 w2244] -> w2233
                  frame False {
                    n730 = for {
                      tunnel: string[] ["START TIMER", "COLOUR PROCESSING", ""] ("element") -> [w2240] mode=indexing
                      shift-right: [w2242] -> w2239
                      shift-left: w2238 -> [w2241]
                      n731 = Enqueue Element(queue=w2241, element=w2240) -> (queue out=w2242:refnum<queue>)  [unwired: 2 in, 2 out]
                    }
                  }
                  frame True {
                    n732 = for {
                      shift-right: [w2247] -> w2244
                      shift-left: w2245 -> [w2248]
                      tunnel: string[] ["DISPOSE BUFFERS", "CLOSE CAM", "RESET ENCODERS", "RESET YAW", "RESET FLAGS"] -> [w2246] mode=indexing
                      n733 = Enqueue Element(queue=w2248, element=w2246) -> (queue out=w2247:refnum<queue>)  [unwired: 2 in, 2 out]
                    }
                  }
                }
                n734 = Or(x=w2228, y=w2227) -> (x .or. y?=w2226:bool)
                n735 = Select(t=State_Type_Definitions."True Stop" ("Enum"), s=w2227, f=State_Type_Definitions."Task 9H: MOVE RIGHT" ("Enum")) -> (s? t:f=w2229:T16)
                n736 = Select(t=w2229, s=w2226, f=State_Type_Definitions."Task 9G: PROCESS COLOUR" ("Enum")) -> (s? t:f=w2235:T16)
              }
              frame "Exit" {
                n737 = for {
                  shift-right: [w2255] -> w2252
                  shift-left: w2251 -> [w2256]
                  tunnel: string[] ["STOP", "RESET ENCODERS", "RESET YAW", "ARDUINO MODE 0"] -> [w2254] mode=indexing
                  n738 = Enqueue Element(queue=w2256, element=w2254) -> (queue out=w2255:refnum<queue>)  [unwired: 2 in, 2 out]
                }
              }
            }
          }
          frame "Task 9H: MOVE RIGHT" {
            # ">> Item Selection Bias >>"
            # ">>> Motor control cluster >>>"
            # ">>> yStepper command>>>"
            n739 = Dequeue Element(queue=w2266, timeout in ms (-1)=w2267, error in (no error)=w2268) -> (element=w2270:T8)  [unwired: 3 out]
            n740 = Greater?(x=w2258, y=50.0) -> (0:w2259:bool)
            n741 = And(x=w2260, y=w2259) -> (x .and. y?=w2261:bool)
            n742 = case shown="\"Start Task 1\", Default" w2270 {
              tunnel: w2261 -> [w2276 _]
              tunnel: [w2283 State_Type_Definitions."True Stop" ("Enum")] -> w2263
              tunnel: w2269 -> [w2275 _]
              tunnel: w2265 -> [w2282 w2299]
              tunnel: [w2281 w2300] -> w2264
              tunnel: [State_Type_Definitions."Idle" ("Enum") State_Type_Definitions."Shutdown" ("Enum")] -> w2262
              frame "Start Task 1", Default {
                n743 = case shown="False" w2276 {
                  tunnel: w2282 -> [w2286 w2293]
                  tunnel: [w2287 w2292] -> w2281
                  frame False {
                    n744 = for {
                      tunnel: string[] ["READ LINE SENSOR", "READ NAVX", "RIGHT", "READ ENCODERS"] ("element") -> [w2288] mode=indexing
                      shift-right: [w2290] -> w2287
                      shift-left: w2286 -> [w2289]
                      n745 = Enqueue Element(queue=w2289, element=w2288) -> (queue out=w2290:refnum<queue>)  [unwired: 2 in, 2 out]
                    }
                  }
                  frame True {
                    n746 = for {
                      shift-right: [w2295] -> w2292
                      shift-left: w2293 -> [w2296]
                      tunnel: string[] ["STOP", "RESET ENCODERS", "RESET YAW", "OPEN LIFE CAM", "SET TIMER 2", "RESET FLAGS"] -> [w2294] mode=indexing
                      n747 = Enqueue Element(queue=w2296, element=w2294) -> (queue out=w2295:refnum<queue>)  [unwired: 2 in, 2 out]
                    }
                  }
                }
                n748 = Or(x=w2276, y=w2275) -> (x .or. y?=w2274:bool)
                n749 = Select(t=State_Type_Definitions."True Stop" ("Enum"), s=w2275, f=State_Type_Definitions."Task 9I: SCAN IMAGE" ("Enum")) -> (s? t:f=w2277:T16)
                n750 = Select(t=w2277, s=w2274, f=State_Type_Definitions."Task 9H: MOVE RIGHT" ("Enum")) -> (s? t:f=w2283:T16)
              }
              frame "Exit" {
                n751 = for {
                  shift-right: [w2303] -> w2300
                  shift-left: w2299 -> [w2304]
                  tunnel: string[] ["STOP", "RESET ENCODERS", "RESET YAW", "ARDUINO MODE 0"] -> [w2302] mode=indexing
                  n752 = Enqueue Element(queue=w2304, element=w2302) -> (queue out=w2303:refnum<queue>)  [unwired: 2 in, 2 out]
                }
              }
            }
          }
          frame "Task 9I: SCAN IMAGE" {
            # ">> Item Selection Bias >>"
            n753 = Dequeue Element(queue=w2306, timeout in ms (-1)=w2307, error in (no error)=w2308) -> (element=w2314:T8)  [unwired: 3 out]
            n754 = case shown="\"Start Task 1\", Default" w2314 {
              tunnel: w2305 -> [w2320 _]